vi "UHR-Fleezers Control (host) - 10.7.vi"() -> ()   [LabVIEW 2010] (continued)
        n1245 = event-data() -> ("CtlRef"=w4736:refnum<vi>)  [unwired: 6 out]
        n1246 = control-ref of="Trap Delta (MHz)"() -> (w4735:refnum<vi>)
        n1247 = Equal?(x=w4735, y=w4736) -> (x = y?=w4734:bool)
        n1248 = case shown="False" "Oscillate Set 2" {
          tunnel: w4739 -> [w4759 _]
          tunnel: [w4758 w4762] -> w4738
          tunnel: w4737 -> [w4757 w4762]
          tunnel: w4734 -> [w4742 _]
          frame False {
            n1249 = local read "BD 1 Frequency 2 (MHz)"() -> (w4746:dbl)
            n1250 = local read "BD 1 Frequency 1 (MHz)"() -> (w4744:dbl)
            n1251 = Subtract(x=w4746, y="Trap Delta (MHz)") -> (x-y=w4743:dbl)
            n1252 = Select(t=w4743, s=w4742, f=w4744) -> (s? t:f=w4741:dbl)
            n1253 = local read "Y RF Frequency Limits (MHz)"() -> (w4747:T16)
            n1254 = local read "X RF Frequency Limits (MHz)"() -> (w4748:T16)
            n1255 = local read "BD 1 Frequency 3 (MHz)"() -> (w4760:dbl)
            n1256 = local write "BD 1 Frequency 1 (MHz)"(w4741) -> ()
            n1257 = local read "BD 2 Frequency 1 (MHz)"() -> (w4751:dbl)
            n1258 = local read "BD 2 Frequency 2 (MHz)"() -> (w4750:dbl)
            n1259 = local read "BD 2 Frequency 3 (MHz)"() -> (w4761:dbl)
            n1260 = call "set RF board frequency - interlace.vi"("Board 2 Frequency Limits"=w4747, "Board 1 Frequency Limits"=w4748, "error in"=w4757, "FPGA VI Reference In"=w4759, "Board 2 Frequency 3 (MHz)"=w4761, "Board 1 Frequency 3 (MHz)"=w4760, "Board 2 Frequency 2 (MHz)"=w4750, "Board 2 Frequency 1 (MHz)"=w4751, "Board 1 Frequency 2 (MHz)"=w4746, "Board 1 Frequency 1  (MHz)"=w4741) -> ("error out"=w4758:errorcluster)  [unwired: 1 out]
            n1261 = Subtract(x=w4751, y=w4750) -> (x-y=w4755:dbl)
            n1262 = Subtract(x=w4741, y=w4746) -> (x-y=w4756:dbl)
            n1263 = Square(x=w4755) -> (x^2=w4753:dbl)
            n1264 = Square(x=w4756) -> (x^2=w4754:dbl)
            n1265 = Add(x=w4754, y=w4753) -> (x+y=w4752:dbl)
            n1266 = Square Root(x=w4752) -> (sqrt(x)=w4749:dbl)
            n1267 = local write "Trap Delta (MHz)"(w4749) -> ()
            n1268 = property on="Initial delta (MHz)" class="DigNum (strict)"("Val(Sgnl)"=w4749) -> ()  [unwired: 2 in, 2 out]
          }
          frame True {
          }
        }
      }
      event "Round T1 X": Value Change {
        n1269 = event-data() -> ()  [unwired: 7 out]
        n1270 = local read "BD 1 Frequency 1 (MHz)"() -> (w4765:dbl)
        n1271 = Round To Nearest(number=w4765) -> (nearest integer value=w4764:dbl)
        n1272 = property on="BD 1 Frequency 1 (MHz)" class="DigNum (strict)"("Val(Sgnl)"=w4764) -> ()  [unwired: 2 in, 2 out]
      }
      event "Restart RF": Value Change {
        n1273 = event-data() -> ()  [unwired: 7 out]
        n1274 = xnode "Read/Write Control"("FPGA VI Reference In"=w4803, "error in"=w4798, "FPGA Controls  RF Box"=FALSE) -> ("FPGA VI Reference Out"=w4802:T19, "error out"=w4797:errorcluster)
        n1275 = local read "Y RF Amplitude Limits (%)"() -> (w4778:T16)
        n1276 = local read "X RF Amplitude Limits (%)"() -> (w4779:T16)
        n1277 = local read "X RF Frequency Limits (MHz)"() -> (w4781:T16)
        n1278 = local read "Y RF Frequency Limits (MHz)"() -> (w4780:T16)
        n1279 = xnode "Read/Write Control"("FPGA VI Reference In"=w4802, "error in"=w4797, "Direct RF Box  Communication"=TRUE) -> ("FPGA VI Reference Out"=w4801:T19, "error out"=w4796:errorcluster)
        n1280 = local read "BD 2 Frequency 3 (MHz)"() -> (w4788:dbl)
        n1281 = local read "BD 2 Frequency 2 (MHz)"() -> (w4789:dbl)
        n1282 = local read "BD 1 Frequency 3 (MHz)"() -> (w4792:dbl)
        n1283 = local read "BD 1 Frequency 1 (MHz)"() -> (w4793:dbl)
        n1284 = local read "BD 2 Frequency 1 (MHz)"() -> (w4790:dbl)
        n1285 = local read "BD 1 Frequency 2 (MHz)"() -> (w4791:dbl)
        n1286 = call "Initialize RF boards - interlace 3.vi"("error in"=w4796, "FPGA VI Reference In"=w4801) -> ("error out"=w4795:errorcluster, "FPGA VI Reference Out"=w4800:T19)
        n1287 = local read "BD 2 Amplitude 2 (%)"() -> (w4783:dbl)
        n1288 = local read "BD 2 Amplitude 1 (%)"() -> (w4784:dbl)
        n1289 = local read "BD 2 Amplitude 3 (%)"() -> (w4782:dbl)
        n1290 = local read "BD 1 Amplitude 3 (%)"() -> (w4787:dbl)
        n1291 = local read "BD 1 Amplitude 1 (%)"() -> (w4786:dbl)
        n1292 = local read "BD 1 Amplitude 2 (%)"() -> (w4785:dbl)
        n1293 = call "set RF board frequency - interlace.vi"("Board 2 Frequency Limits"=w4780, "Board 1 Frequency Limits"=w4781, "error in"=w4795, "FPGA VI Reference In"=w4800, "Board 2 Frequency 3 (MHz)"=w4788, "Board 1 Frequency 3 (MHz)"=w4792, "Board 2 Frequency 2 (MHz)"=w4789, "Board 2 Frequency 1 (MHz)"=w4790, "Board 1 Frequency 2 (MHz)"=w4791, "Board 1 Frequency 1  (MHz)"=w4793) -> ("error out"=w4794:errorcluster, "FPGA VI Reference Out"=w4799:T19)
        n1294 = call "set RF board amplitude - interlace.vi"("Board 2 Amplitude Limits"=w4778, "Board 1 Amplitude Limits"=w4779, "error in"=w4794, "FPGA VI Reference In"=w4799, "Board 2 Amplitude 3 (%)"=w4782, "Board 1 Amplitude 3 (%)"=w4787, "Board 2 Amplitude 2 (%)"=w4783, "Board 2 Amplitude 1 (%)"=w4784, "Board 1 Amplitude 2 (%)"=w4785, "Board 1 Amplitude 1 (%)"=w4786) -> ("error out"=w4771:errorcluster, "FPGA VI Reference Out"=w4775:T19)
        n1295 = xnode "Read/Write Control"("FPGA VI Reference In"=w4775, "error in"=w4771, "Direct RF Box  Communication"=FALSE) -> ("FPGA VI Reference Out"=w4774:T19, "error out"=w4773:errorcluster)
        n1296 = flat-sequence {
          tunnel: w4773 -> [w4804]
          tunnel: [w4804] -> w4772
          frame #0 {
            n1297 = Wait (ms)(milliseconds to wait=u32 50) -> ()  [unwired: 1 out]
          }
        }
        n1298 = xnode "Read/Write Control"("FPGA VI Reference In"=w4774, "error in"=w4772, "FPGA Controls  RF Box"=TRUE) -> ("error out"=w4767:errorcluster)  [unwired: 1 out]
        n1299 = property on="Restart RF" class="Bool (strict)"(error in=w4767, "Value"=FALSE ("Restart RF")) -> (error out=w4766:errorcluster)  [unwired: 1 in, 1 out]
      }
      event "Round T2 X": Value Change {
        n1300 = event-data() -> ()  [unwired: 7 out]
        n1301 = local read "BD 1 Frequency 2 (MHz)"() -> (w4959:dbl)
        n1302 = Round To Nearest(number=w4959) -> (nearest integer value=w4958:dbl)
        n1303 = property on="BD 1 Frequency 2 (MHz)" class="DigNum (strict)"("Val(Sgnl)"=w4958) -> ()  [unwired: 2 in, 2 out]
      }
      event "Stop All": Value Change {
        n1304 = event-data() -> ()  [unwired: 7 out]
        n1305 = call "hamilton_controller.vi"("action"=T23."DISCONNECT") -> ()  [unwired: 10 in, 1 out]
        n1306 = local read "Stop All"() -> (w4962:bool)
      }
      event "Delayed Interlace Start": Value Change {
        n1307 = event-data() -> ()  [unwired: 7 out]
        n1308 = flat-sequence {
          frame #0 {
            n1309 = Multiply(x="Delay to Interlace (s)", y=1000.0) -> (x*y=w4965:dbl)
            n1310 = Wait (ms)(milliseconds to wait=w4965) -> ()  [unwired: 1 out]
          }
          frame #1 {
            n1311 = property on="Green laser mode" class="RadioBtnsControl (strict)"("Val(Sgnl)"=enum32{"Laser ON", "Laser OFF", "Interlace"}."Interlace" ("Value (Signaling)")) -> ()  [unwired: 2 in, 2 out]
          }
        }
      }
      event "BD 1 Amplitude 1 (%)", "BD 1 Amplitude 2 (%)", "BD 1 Amplitude 3 (%)", "BD 2 Amplitude 1 (%)", "BD 2 Amplitude 2 (%)", "BD 2 Amplitude 3 (%)", "Trap 1 ON", "Trap 2 ON", "Trap 3 ON", "Feedback On/Off", "All FB On/Off": Value Change {
        w4989 = i16 1 ("f")
        n1312 = event-data() -> ()  [unwired: 7 out]
        n1313 = local write "Trap 1 (ON/OFF)"("Trap 1 ON") -> ()
        n1314 = local write "Trap 2 (ON/OFF)"("Trap 2 ON") -> ()
        n1315 = Boolean To (0,1)(Boolean="Trap 3 ON") -> (0, 1=w4990:i16)
        n1316 = Boolean To (0,1)(Boolean="Trap 1 ON") -> (0, 1=w4991:i16)
        n1317 = Boolean To (0,1)(Boolean="Trap 2 ON") -> (0, 1=w4992:i16)
        n1318 = Select(t=w4992, s="Trap ON/OFF X or Y Amp?", f=w4989) -> (s? t:f=w4987:i16)
        n1319 = Select(t=w4991, s="Trap ON/OFF X or Y Amp?", f=w4989) -> (s? t:f=w4988:i16)
        n1320 = Select(t=w4990, s="Trap ON/OFF X or Y Amp?", f=w4989) -> (s? t:f=w4986:i16)
        n1321 = Select(t=w4989, s="Trap ON/OFF X or Y Amp?", f=w4992) -> (s? t:f=w4984:i16)
        n1322 = Select(t=w4989, s="Trap ON/OFF X or Y Amp?", f=w4991) -> (s? t:f=w4985:i16)
        n1323 = Select(t=w4989, s="Trap ON/OFF X or Y Amp?", f=w4990) -> (s? t:f=w4983:i16)
        n1324 = And(x="All FB On/Off", y="Feedback On/Off") -> (x .and. y?=w4981:cluster{"Set 1":bool, "Set 2":bool})
        n1325 = local read "BD 1 Amplitude 1 (%)"() -> (w5001:dbl)
        n1326 = local read "BD 1 Amplitude 2 (%)"() -> (w5000:dbl)
        n1327 = local read "BD 1 Amplitude 3 (%)"() -> (w4999:dbl)
        n1328 = Unbundle By Name(w4981) -> ("Set 1"=w4976:bool, "Set 2"=w4973:bool)
        n1329 = local read "Y RF Amplitude Limits (%)"() -> (w4969:T16)
        n1330 = local read "X RF Amplitude Limits (%)"() -> (w4970:T16)
        n1331 = local read "BD 2 Amplitude 1 (%)"() -> (w5002:dbl)
        n1332 = local read "BD 2 Amplitude 2 (%)"() -> (w5003:dbl)
        n1333 = local read "BD 2 Amplitude 3 (%)"() -> (w5004:dbl)
        n1334 = And(x="Trap 2 ON", y=w4973) -> (x .and. y?=w4971:bool)
        n1335 = And(x="Trap 1 ON", y=w4976) -> (x .and. y?=w4974:bool)
        n1336 = Multiply(x=w4988, y=w5001) -> (x*y=w4996:dbl)
        n1337 = Multiply(x=w5000, y=w4987) -> (x*y=w4994:dbl)
        n1338 = Multiply(x=w4999, y=w4986) -> (x*y=w4995:dbl)
        n1339 = Multiply(x=w5002, y=w4985) -> (x*y=w5005:dbl)
        n1340 = Multiply(x=w5003, y=w4984) -> (x*y=w5006:dbl)
        n1341 = Multiply(x=w5004, y=w4983) -> (x*y=w5007:dbl)
        n1342 = call "set RF board amplitude - interlace.vi"("Board 2 Amplitude Limits"=w4969, "Board 1 Amplitude Limits"=w4970, "error in"=w4997, "FPGA VI Reference In"=w4998, "Board 2 Amplitude 3 (%)"=w5007, "Board 1 Amplitude 3 (%)"=w4995, "Board 2 Amplitude 2 (%)"=w5006, "Board 2 Amplitude 1 (%)"=w5005, "Board 1 Amplitude 2 (%)"=w4994, "Board 1 Amplitude 1 (%)"=w4996) -> ("error out"=w4978:errorcluster, "FPGA VI Reference Out"=w4979:T19)
        n1343 = xnode "Read/Write Control"("FPGA VI Reference In"=w4979, "error in"=w4978, "FB On/Off Set 1"=w4974, "FB On/Off Set 2"=w4971) -> ("error out"=w4977:errorcluster)  [unwired: 1 out]
      }
      event "Load parameters": Value Change {
        n1344 = event-data() -> ()  [unwired: 7 out]
        n1345 = property on="Saved AOD Raster Scan Parameter Sets" class="Arr (strict)"() -> ("Index Values"=w5077:u32[])  [unwired: 2 in, 2 out]
        n1346 = Index Array(array=w5077, index=0) -> (element=w5074:u32)
        n1347 = local write "Load parameters"(FALSE ("Load parameters")) -> ()
        n1348 = Index Array(array="Saved AOD Raster Scan Parameter Sets", index=w5074) -> (element=w5073:T48)
        n1349 = Unbundle By Name(w5073) -> ("Scan Range AOD (nm) 2"=w5072:dbl, "Step Size AOD (nm) 2"=w5071:dbl, "Scan Speed AOD (nm/s) 2"=w5070:dbl, "Number of scans (AOD) 2"=w5069:u16)
        n1350 = flat-sequence {
          tunnel: w5072 -> [w5080]
          tunnel: w5071 -> [w5079]
          tunnel: w5070 -> [w5078]
          tunnel: w5069 -> [w5081]
          frame #0 {
            n1351 = local write "Scan Speed (nm/s)"(w5078) -> ()
            n1352 = local write "Scan Range (nm)"(w5080) -> ()
            n1353 = local write "Step Size (nm)"(w5079) -> ()
          }
          frame #1 {
            n1354 = property on="Number of F/B Scans (AOD)" class="DigNum (strict)"("Val(Sgnl)"=w5081) -> ()  [unwired: 2 in, 2 out]
          }
        }
      }
      event "Trap 1 (ON/OFF)", "Trap 2 (ON/OFF)": Value Change {
        n1355 = event-data() -> ()  [unwired: 7 out]
        n1356 = property on="Trap 2 ON" class="Bool (strict)"("Val(Sgnl)"="Trap 2 (ON/OFF)") -> ()  [unwired: 2 in, 2 out]
        n1357 = property on="Trap 1 ON" class="Bool (strict)"("Val(Sgnl)"="Trap 1 (ON/OFF)") -> ()  [unwired: 2 in, 2 out]
      }
      event "DIO count 1 (ticks)", "DIO count 2 (ticks)", "DIO count 3 (ticks)", "Interlace", "Number Interlace Sets", "Not-Interlacing Set": Value Change {
        n1358 = event-data() -> ()  [unwired: 7 out]
        n1359 = local read "DIO count 3 (ticks)"() -> (w5094:u32)
        n1360 = local read "DIO count 1 (ticks)"() -> (w5096:u32)
        n1361 = local read "DIO count 2 (ticks)"() -> (w5095:u32)
        n1362 = To Unsigned Byte Integer(number="Not-Interlacing Set") -> (unsigned 8bit integer=w5085:u8)
        n1363 = Add(x=w5085, y=u8 1) -> (x+y=w5089:u8)
        n1364 = xnode "Read/Write Control"("FPGA VI Reference In"=w5100, "error in"=w5098, "DIO count 1 (ticks)"=w5096, "DIO count 2 (ticks)"=w5095, "DIO count 3 (ticks)"=w5094, "Interlace ON/OFF"="Interlace", "Number Interlace Cycles"="Number Interlace Sets", "Interlace Off Parameters"=w5089) -> ("error out"=w5099:errorcluster)  [unwired: 1 out]
        n1365 = Build Array(w5096, w5095, w5094) -> (w5087:u32[])
        n1366 = Split 1D Array(array=w5087, index="Number Interlace Sets") -> (first subarray=w5097:u32[])  [unwired: 1 out]
        n1367 = Index Array(array=w5087, index=w5085) -> (element=w5086:u32)
        n1368 = Add Array Elements(numeric array=w5097) -> (sum=w5091:u32)
        n1369 = Select(t=w5091, s="Interlace", f=w5086) -> (s? t:f=→"Total Counts (ticks)":u32)
      }
      event "Reset Feedback": Value Change {
        n1370 = event-data() -> ()  [unwired: 7 out]
        n1371 = Unbundle By Name("Reset Feedback") -> ("Set 1"=w5242:bool, "Set 2"=w5241:bool)
        n1372 = xnode "Read/Write Control"("FPGA VI Reference In"=w5244, "error in"=w5239, "FB Reset Set 1"=w5242, "FB Reset Set 2"=w5241) -> ("error out"=w5240:errorcluster)  [unwired: 1 out]
      }
      event "PID Gains": Value Change {
        n1373 = event-data() -> ()  [unwired: 7 out]
        n1374 = Unbundle By Name("PID Gains") -> ("Set 1"=w5307:T14, "Set 2"=w5306:T14)
        n1375 = xnode "Read/Write Control"("FPGA VI Reference In"=w5308, "error in"=w5304, "FB Gains Set 1"=w5307, "FB Gains Set 2"=w5306) -> ("error out"=w5305:errorcluster)  [unwired: 1 out]
      }
      event "AI2 to Setpoint", "Trap Intensity\nSetpoints (V)": Value Change {
        n1376 = event-data() -> ()  [unwired: 7 out]
        n1377 = xnode "Read/Write Control"("FPGA VI Reference In"=w5383, "error in"=w5379) -> ("FPGA VI Reference Out"=w5382:T19, "error out"=w5381:errorcluster, "AI2 Y Sum Set 1"=w5390:i16, "AI2 Y Sum Set 2"=w5389:i16)
        n1378 = Cluster To Array(cluster="AI2 to Setpoint") -> (array=w5393:bool[])
        n1379 = local read "AI2 (V)"() -> (w5391:cluster{"Set 1":dbl, "Set 2":dbl})
        n1380 = Or Array Elements(Boolean array=w5393) -> (logical OR=w5394:bool)
        n1381 = Bundle By Name(cluster=w5391, "Set 1"=w5390, "Set 2"=w5389) -> (w5388:cluster{"Set 1":dbl, "Set 2":dbl})
        n1382 = Divide(x=w5388, y=3276.7) -> (x/y=w5387:cluster{"Set 1":dbl, "Set 2":dbl})
        "AI2 (V)" <- w5387
        n1383 = case shown="True" w5394 {
          tunnel: [w5458 w5475] -> w5386
          tunnel: "AI2 to Setpoint" -> [_ w5471]
          tunnel: "Trap Intensity\nSetpoints (V)" -> [w5459 w5474]
          tunnel: w5387 -> [_ w5468]
          frame False {
            n1384 = Multiply(x=3276.7, y=w5459) -> (x*y=w5460:cluster{"Set 1":dbl, "Set 2":dbl})
            n1385 = To Word Integer(number=w5460) -> (16bit integer=w5458:cluster{"Set 1":i16, "Set 2":i16})
          }
          frame True {
            n1386 = Unbundle By Name(w5468) -> ("Set 1"=w5467:dbl, "Set 2"=w5466:dbl)
            n1387 = Unbundle By Name(w5474) -> ("Set 1"=w5473:dbl, "Set 2"=w5472:dbl)
            n1388 = Unbundle By Name(w5471) -> ("Set 1"=w5470:bool, "Set 2"=w5469:bool)
            n1389 = Select(t=w5467, s=w5470, f=w5473) -> (s? t:f=w5465:dbl)
            n1390 = Select(t=w5466, s=w5469, f=w5472) -> (s? t:f=w5464:dbl)
            n1391 = Bundle By Name(cluster=w5474, "Set 1"=w5465, "Set 2"=w5464) -> (w5462:cluster{"Set 1":dbl, "Set 2":dbl})
            n1392 = local write "Trap Intensity\nSetpoints (V)"(w5462) -> ()
            n1393 = Multiply(x=3276.7, y=w5462) -> (x*y=w5463:cluster{"Set 1":dbl, "Set 2":dbl})
            n1394 = To Word Integer(number=w5463) -> (16bit integer=w5475:cluster{"Set 1":i16, "Set 2":i16})
          }
        }
        n1395 = Unbundle By Name(w5386) -> ("Set 1"=w5385:i16, "Set 2"=w5384:i16)
        n1396 = xnode "Read/Write Control"("FPGA VI Reference In"=w5382, "error in"=w5381, "FB Setpoint Set 1"=w5385, "FB Setpoint Set 2"=w5384) -> ("error out"=w5380:errorcluster)  [unwired: 1 out]
      }
      event "Invert GI": Value Change {
        n1397 = event-data() -> ()  [unwired: 7 out]
        n1398 = xnode "Read/Write Control"("FPGA VI Reference In"=w5537, "error in"=w5535, "Invert GI"="Invert GI", "Invert GI 2"="Invert GI") -> ("error out"=w5536:errorcluster)  [unwired: 1 out]
      }
      event "Green FB Setpoint (mV)", "Green FB Gains", "Green FB On/Off", "Current When FB OFF (%)", "Green int current ON count adj": Value Change {
        n1399 = event-data() -> ()  [unwired: 7 out]
        n1400 = local read "Green FB Setpoint (mV)"() -> (w5603:dbl)
        n1401 = local read "Current When FB OFF (%)"() -> (w5606:dbl)
        n1402 = Multiply(x=w5603, y=3.2767) -> (x*y=w5602:dbl)
        n1403 = Multiply(x=w5606, y=655.35) -> (x*y=w5607:dbl)
        n1404 = To Unsigned Word Integer(number=w5607) -> (unsigned 16bit integer=w5605:u16)
        n1405 = local read "Green int current ON count adj"() -> (w5610:u32)
        n1406 = local read "Green FB Gains"() -> (w5609:T14)
        n1407 = local read "Green Laser ON/Interlacing"() -> (w5600:bool)
        n1408 = local read "Green laser mode"() -> (w5599:enum32{"Laser ON", "Laser OFF", "Interlace"})
        n1409 = local read "Green FB On/Off"() -> (w5611:bool)
        n1410 = Equal?(x=w5599, y=enum32{"Laser ON", "Laser OFF", "Interlace"}."Interlace") -> (x = y?=w5597:bool)
        n1411 = Compound Arithmetic op=AND(w5597, w5611, w5600) -> (w5601:bool)
        n1412 = xnode "Read/Write Control"("FPGA VI Reference In"=w5614, "error in"=w5613, "Green FB Setpoint"=w5602, "Green FB On/Off"=w5601, "Current Out"=w5605, "Green int current ON count adj"=w5610, "Green FB Gains"=w5609) -> ("error out"=w5612:errorcluster)  [unwired: 1 out]
      }
      event "Green laser mode", "Green Laser ON/Interlacing": Value Change {
        n1413 = event-data() -> ()  [unwired: 7 out]
        n1414 = case shown="True" "Green Laser ON/Interlacing" {
          tunnel: "Green laser mode" -> [_ w5752]
          tunnel: [enum32{"Laser ON", "Laser OFF", "Interlace"}."Laser OFF" ("Green laser mode") w5752] -> w5740
          tunnel: [FALSE w5748] -> w5739
          frame False {
          }
          frame True {
            n1415 = local read "Green FB On/Off"() -> (w5749:bool)
            n1416 = Equal?(x=w5752, y=enum32{"Laser ON", "Laser OFF", "Interlace"}."Interlace") -> (x = y?=w5750:bool)
            n1417 = And(x=w5750, y=w5749) -> (x .and. y?=w5748:bool)
          }
        }
        n1418 = xnode "Read/Write Control"("FPGA VI Reference In"=w5745, "error in"=w5743, "Operating Mode"=w5740, "Operating Mode 2"=w5740, "Green FB On/Off"=w5739) -> ("error out"=w5744:errorcluster)  [unwired: 1 out]
      }
      event "Use mouse to move stage\n(press mouse wheel to quit)": Value Change {
        n1419 = event-data() -> ()  [unwired: 7 out]
      }
      event "- phase (APD 1 Gate)", "+ phase (APD 1 Gate)": Value Change {
        n1420 = event-data() -> ()  [unwired: 7 out]
        n1421 = local read "Phase Adj. (APD 1 Gate)"() -> (w5831:i16)
        n1422 = Negate(x=w5831) -> (-x=w5839:i16)
        n1423 = Select(t=w5839, s="- phase (APD 1 Gate)", f=w5831) -> (s? t:f=w5838:i16)
        n1424 = Or(x="- phase (APD 1 Gate)", y="+ phase (APD 1 Gate)") -> (x .or. y?=w5834:bool)
        n1425 = xnode "Read/Write Control"("FPGA VI Reference In"=w5841, "error in"=w5840, "Phase count adjustment (APD 1 Gate)"=w5838) -> ("FPGA VI Reference Out"=w5836:T19, "error out"=w5837:errorcluster)
        n1426 = xnode "Read/Write Control"("FPGA VI Reference In"=w5836, "error in"=w5837, "+ phase (APD 1 Gate)"=w5834) -> ("error out"=w5835:errorcluster)  [unwired: 1 out]
      }
      event "+ phase (APD 2 Gate)", "- phase (APD 2 Gate)": Value Change {
        n1427 = event-data() -> ()  [unwired: 7 out]
        n1428 = local read "Phase Adj. (APD 2 Gate)"() -> (w5917:i16)
        n1429 = Negate(x=w5917) -> (-x=w5925:i16)
        n1430 = Select(t=w5925, s="- phase (APD 2 Gate)", f=w5917) -> (s? t:f=w5924:i16)
        n1431 = Or(x="- phase (APD 2 Gate)", y="+ phase (APD 2 Gate)") -> (x .or. y?=w5920:bool)
        n1432 = xnode "Read/Write Control"("FPGA VI Reference In"=w5927, "error in"=w5926, "Phase count adjustment (APD 2 Gate)"=w5924) -> ("FPGA VI Reference Out"=w5922:T19, "error out"=w5923:errorcluster)
        n1433 = xnode "Read/Write Control"("FPGA VI Reference In"=w5922, "error in"=w5923, "+ phase (APD 2 Gate)"=w5920) -> ("error out"=w5921:errorcluster)  [unwired: 1 out]
      }
      event "Phase Adj. (APD Acq)", "+ phase (APD Acq)", "- phase (APD Acq)": Value Change {
        n1434 = event-data() -> ()  [unwired: 7 out]
        n1435 = local read "Phase Adj. (APD Acq)"() -> (w6005:i16)
        n1436 = Negate(x=w6005) -> (-x=w6011:i16)
        n1437 = Select(t=w6011, s="+ phase (APD Acq)", f=w6005) -> (s? t:f=w6010:i16)
        n1438 = Or(x="+ phase (APD Acq)", y="- phase (APD Acq)") -> (x .or. y?=w6006:bool)
        n1439 = xnode "Read/Write Control"("FPGA VI Reference In"=w6013, "error in"=w6012, "Phase Count Adjustment (APD Acq)"=w6010) -> ("FPGA VI Reference Out"=w6008:T19, "error out"=w6009:errorcluster)
        n1440 = xnode "Read/Write Control"("FPGA VI Reference In"=w6008, "error in"=w6009, "+ phase (APD Acq)"=w6006) -> ("error out"=w6007:errorcluster)  [unwired: 1 out]
      }
      event "Phase adj. (GI)", "+ phase (GI)", "- phase (GI)": Value Change {
        n1441 = event-data() -> ()  [unwired: 7 out]
        n1442 = Negate(x="Phase adj. (GI)") -> (-x=w6097:i16)
        n1443 = Select(t=w6097, s="+ phase (GI)", f="Phase adj. (GI)") -> (s? t:f=w6096:i16)
        n1444 = Or(x="+ phase (GI)", y="- phase (GI)") -> (x .or. y?=w6092:bool)
        n1445 = xnode "Read/Write Control"("FPGA VI Reference In"=w6099, "error in"=w6098, "Phase count adjustment (GI)"=w6096) -> ("FPGA VI Reference Out"=w6094:T19, "error out"=w6095:errorcluster)
        n1446 = xnode "Read/Write Control"("FPGA VI Reference In"=w6094, "error in"=w6095, "+ phase (GI)"=w6092) -> ("error out"=w6093:errorcluster)  [unwired: 1 out]
      }
      event "Phase adj. (GI) 2", "+ phase (GI) 2", "- phase (GI) 2": Value Change {
        n1447 = event-data() -> ()  [unwired: 7 out]
        n1448 = Negate(x="Phase adj. (GI) 2") -> (-x=w6183:i16)
        n1449 = Select(t=w6183, s="+ phase (GI) 2", f="Phase adj. (GI) 2") -> (s? t:f=w6182:i16)
        n1450 = Or(x="+ phase (GI) 2", y="- phase (GI) 2") -> (x .or. y?=w6178:bool)
        n1451 = xnode "Read/Write Control"("FPGA VI Reference In"=w6185, "error in"=w6184, "Phase count adjustment (GI) 2"=w6182) -> ("FPGA VI Reference Out"=w6180:T19, "error out"=w6181:errorcluster)
        n1452 = xnode "Read/Write Control"("FPGA VI Reference In"=w6180, "error in"=w6181, "+ phase (GI) 2"=w6178) -> ("error out"=w6179:errorcluster)  [unwired: 1 out]
      }
      event "Phase adj. (Green FB)", "- phase (Green FB)", "+ phase (Green FB)": Value Change {
        n1453 = event-data() -> ()  [unwired: 7 out]
        n1454 = Negate(x="Phase adj. (Green FB)") -> (-x=w6269:i16)
        n1455 = Select(t=w6269, s="+ phase (Green FB)", f="Phase adj. (Green FB)") -> (s? t:f=w6268:i16)
        n1456 = Or(x="+ phase (Green FB)", y="- phase (Green FB)") -> (x .or. y?=w6264:bool)
        n1457 = xnode "Read/Write Control"("FPGA VI Reference In"=w6271, "error in"=w6270, "Phase count adjustment (Green FB)"=w6268) -> ("FPGA VI Reference Out"=w6266:T19, "error out"=w6267:errorcluster)
        n1458 = xnode "Read/Write Control"("FPGA VI Reference In"=w6266, "error in"=w6267, "+ phase (Green FB)"=w6264) -> ("error out"=w6265:errorcluster)  [unwired: 1 out]
      }
      event "Invert APD Gate", "APD Gate ON Count", "APD Gate OFF Count", "APD Gate", "APD Integration Time (s)", "APD 1 AO Mult.", "APD 2 AO Mult.": Value Change {
        n1459 = event-data() -> ()  [unwired: 7 out]
        n1460 = local read "APD Integration Time (s)"() -> (w6347:dbl)
        n1461 = local read "APD Gate ON Count"() -> (w6360:u32)
        n1462 = local read "APD Gate OFF Count"() -> (w6359:u32)
        n1463 = local read "Invert APD Gate"() -> (w6361:bool)
        n1464 = local read "APD Gate"() -> (w6358:enum32{"ON", "OFF", "Interlace"})
        n1465 = Multiply(x=w6347, y=40000000.0) -> (x*y=w6356:dbl)
        n1466 = Reciprocal(x=w6347) -> (1/x=→"APD Acq Rate (Hz)":dbl)
        n1467 = To Unsigned Long Integer(number=w6356) -> (unsigned 32bit integer=w6355:u32)
        n1468 = local read "DMA Update Period (s)"() -> (w6348:dbl)
        n1469 = Divide(x=w6348, y=w6347) -> (x/y=w6351:dbl)
        n1470 = local read "APD 1 AO Mult."() -> (w6353:i16)
        n1471 = local read "APD 2 AO Mult."() -> (w6352:i16)
        n1472 = Multiply(x=2.0, y=w6351) -> (x*y=w6350:dbl)
        n1473 = local write "APD Samples/FIFO Acq."(w6351) -> ()
        n1474 = local write "APD Elements/DMA read"(w6350) -> ()
        n1475 = xnode "Read/Write Control"("FPGA VI Reference In"=w6364, "error in"=w6363, "Invert APD Gate"=w6361, "APD Gate ON Count"=w6360, "APD Gate OFF Count"=w6359, "APD Acq Rate Count"=w6355, "APD Gate Operating Mode"=w6358, "APD 1 AO scale factor"=w6353, "APD 2 AO scale factor"=w6352) -> ("error out"=w6362:errorcluster)  [unwired: 1 out]
      }
      event "GI Frequency, ON count", "Green FB Count", "GI Frequency, OFF count": Value Change {
        n1476 = event-data() -> ()  [unwired: 7 out]
        n1477 = xnode "Read/Write Control"("FPGA VI Reference In"=w6528, "error in"=w6526, "Green interlace ON count"="GI Frequency, ON count", "Green interlace OFF count"="GI Frequency, OFF count", "Green interlace ON count 2"="GI Frequency, ON count", "Green interlace OFF count 2"="GI Frequency, OFF count", "Green FB Count"="Green FB Count") -> ("error out"=w6527:errorcluster)  [unwired: 1 out]
      }
      event "Number of F/B Scans (AOD)", "Scan Speed (nm/s)", "Scan BD", "Initial delta (MHz)", "Step Size (nm)", "Scan Range (nm)": Value Change {
        w6707 = 123.0  # AOM cal (nm/MHz)
        n1478 = event-data() -> ()  [unwired: 7 out]
        n1479 = local read "BD 1 Frequency 1 (MHz)"() -> (w6690:dbl)
        n1480 = local read "AOM X Cal (nm/MHz)"() -> (w6682:dbl)
        n1481 = local read "X RF Frequency Limits (MHz)"() -> (w6694:T16)
        n1482 = local read "Y RF Frequency Limits (MHz)"() -> (w6691:T16)
        n1483 = local read "BD 2 Frequency 1 (MHz)"() -> (w6696:dbl)
        n1484 = Negate(x="Scan Range (nm)") -> (-x=w6660:dbl)
        n1485 = Divide(x=w6660, y=w6682) -> (x/y=w6664:dbl)
        n1486 = Select(t=w6694, s="Scan BD", f=w6691) -> (s? t:f=w6693:T16)
        n1487 = Select(t=w6690, s="Scan BD", f=w6696) -> (s? t:f=w6695:dbl)
        n1488 = Unbundle By Name(w6693) -> ("Maximum"=w6702:dbl, "Minimum"=w6701:dbl)
        n1489 = Add(x=w6664, y=w6695) -> (x+y=w6699:dbl)
        n1490 = Divide(x=w6660, y="Step Size (nm)") -> (x/y=w6679:dbl)
        n1491 = Divide(x="Step Size (nm)", y=w6682) -> (x/y=w6688:dbl)
        n1492 = Absolute Value(x=w6679) -> (abs(x)=w6663:dbl)
        n1493 = Sign(1:w6660) -> (0:w6661:dbl)
        n1494 = In Range and Coerce(upper limit=w6702, x=w6699, lower limit=w6701) -> (coerced(x)=w6698:dbl, In Range?=w6700:bool)
        n1495 = To Unsigned Quad Integer(1:w6663) -> (0:w6678:u64)
        "Scan steps (AOD)" <- w6678
        n1496 = call "IR AOM freq to word.vi"("Frequency In (MHz)"=w6688) -> ("Frequency Word Out (double)"=w6685:dbl)
        n1497 = Multiply(x=w6661, y=w6685) -> (x*y=w6662:dbl)
        n1498 = Subtract(x=w6699, y=w6698) -> (x-y=w6697:dbl)
        n1499 = To Quad Integer(1:w6662) -> (0:w6684:i64)
        "Incr. int (AOD)" <- w6684
        n1500 = Subtract(x=w6664, y=w6697) -> (x-y=w6683:dbl)
        "Scan Range (MHz)" <- w6683
        n1501 = Select(t=w6664, s=w6700, f=w6683) -> (s? t:f=w6703:dbl)
        n1502 = Multiply(x=w6683, y=w6682) -> (x*y=w6681:dbl)
        n1503 = Decrement(x=w6678) -> (x-1=w6731:u64)
        n1504 = Negate(x=w6681) -> (-x=w6677:dbl)
        n1505 = local write "Scan Range (nm)"(w6677) -> ()
        n1506 = Divide(x=w6703, y=w6731) -> (x/y=w6687:dbl)
        "Scan Increment (MHz)" <- w6687
        n1507 = call "IR AOM freq to word.vi"("Frequency In (MHz)"=w6687) -> ("Frequency Word Out (double)"=w6686:dbl)
        n1508 = Divide(x="Step Size (nm)", y="Scan Speed (nm/s)") -> (x/y=w6674:dbl)
        n1509 = To Quad Integer(1:w6686) -> ()  [unwired: 1 out]
        n1510 = local read "Number Interlace Sets"() -> (w6658:u8)
        n1511 = local read "AI Count (ticks)"() -> (w6659:u32)
        n1512 = local read "Total Counts (ticks)"() -> (w6657:u32)
        n1513 = local read "# Samples/trap"() -> (w6689:u32)
        n1514 = Multiply(x=w6659, y=w6658) -> (x*y=w6656:u32)
        n1515 = Divide(x=w6657, y=w6656) -> (x/y=w6655:dbl)
        n1516 = Select(t=w6690, s="Scan BD", f=w6696) -> (s? t:f=w6728:dbl)
        "Initial freq. (MHz)" <- w6728
        n1517 = Add(x=w6703, y=w6728) -> (x+y=→"Final freq. (MHz)":dbl)
        n1518 = Divide(x=w6657, y=40000000.0) -> (x/y=w6673:dbl)
        n1519 = Divide(x=w6674, y=w6673) -> (x/y=w6672:dbl)
        n1520 = To Unsigned Quad Integer(1:w6672) -> (0:w6647:u64)
        n1521 = Quotient & Remainder(x=w6647, y=u64 2) -> (x-y*floor(x/y)=w6651:u64)  [unwired: 1 out]
        n1522 = Equal?(x=w6651, y=u64 0) -> (x = y?=w6649:bool)
        n1523 = Decrement(x=w6647) -> (x-1=w6648:u64)
        n1524 = Select(t=w6647, s=w6649, f=w6648) -> (s? t:f=w6646:u64)
        "Cycles/step (AOD)" <- w6646
        n1525 = xnode "Read/Write Control"("FPGA VI Reference In"=w6739, "error in"=w6738, "Scan steps"=w6678, "Number of scans"="Number of F/B Scans (AOD)", "Cycles per step"=w6646, "Scan freq.  increment"=w6684, "Scan BD"="Scan BD") -> ("error out"=w6737:errorcluster)  [unwired: 1 out]
        n1526 = Multiply(x=w6678, y=w6646) -> (x*y=w6732:u64)
        n1527 = Multiply(x=w6732, y=u64 2) -> (x*y=w6654:u64)
        n1528 = Multiply(x=w6655, y=w6654) -> (x*y=w6653:dbl)
        "Data points/scan (f/b)" <- w6653
        n1529 = Multiply(x=w6653, y="Number of F/B Scans (AOD)") -> (x*y=w6735:dbl)
        "Data points/scans" <- w6735
        n1530 = Divide(x=w6735, y=w6689) -> (x/y=→"N sets should be saved":dbl)
        n1531 = Multiply(x=w6732, y=w6673) -> (x*y=w6671:dbl)
        "Time/Scan (s) (AOD)" <- w6671
        n1532 = Select(t=w6703, s="Scan BD", f=0.0) -> (s? t:f=w6729:dbl)
        n1533 = Select(t=0.0, s="Scan BD", f=w6703) -> (s? t:f=w6725:dbl)
        n1534 = local read "BD 2 Frequency 2 (MHz)"() -> (w6721:dbl)
        n1535 = local read "BD 1 Frequency 2 (MHz)"() -> (w6724:dbl)
        n1536 = Add(x=w6725, y=w6696) -> (x+y=w6722:dbl)
        n1537 = Add(x=w6690, y=w6729) -> (x+y=w6723:dbl)
        n1538 = Multiply(x=w6671, y=2.0) -> (x*y=w6670:dbl)
        n1539 = Multiply(x=w6670, y="Number of F/B Scans (AOD)") -> (x*y=w6667:dbl)
        n1540 = Divide(x=w6667, y=60.0) -> (x/y=→"Time to Finish All (min)":dbl)
        n1541 = Add(x="Trap 2 Bead Size (nm)", y="Trap 1 Bead Size (nm)") -> (x+y=w6711:dbl)
        n1542 = Divide(x=w6711, y=2.0) -> (x/y=w6705:dbl)
        n1543 = local read "Initial delta (MHz)"() -> (w6708:dbl)
        n1544 = Subtract(x=w6722, y=w6721) -> (x-y=w6719:dbl)
        n1545 = Subtract(x=w6723, y=w6724) -> (x-y=w6720:dbl)
        n1546 = Square(x=w6719) -> (x^2=w6718:dbl)
        n1547 = Square(x=w6720) -> (x^2=w6717:dbl)
        n1548 = Add(x=w6717, y=w6718) -> (x+y=w6716:dbl)
        n1549 = Square Root(x=w6716) -> (sqrt(x)=w6715:dbl)
        "Final delta (MHz)" <- w6715
        n1550 = Multiply(x=w6707, y=w6715) -> (x*y=w6714:dbl)
        n1551 = Multiply(x=w6708, y=w6707) -> (x*y=w6706:dbl)
        n1552 = Subtract(x=w6706, y=w6705) -> (x-y=→"Initial sep (nm)":dbl)
        n1553 = Subtract(x=w6714, y=w6705) -> (x-y=→"Final sep (nm)":dbl)
      }
      event "Freq or Amp switch first", "Swap F1 and F2", "Freq switch delay", "Amp switch delay": Value Change {
        n1554 = event-data() -> ()  [unwired: 7 out]
        n1555 = local read "Freq or Amp switch first"() -> (w6876:bool)
        n1556 = local read "Amp switch delay"() -> (w6877:u16)
        n1557 = local read "Freq switch delay"() -> (w6879:u16)
        n1558 = local read "Swap F1 and F2"() -> (w6878:bool)
        n1559 = xnode "Read/Write Control"("FPGA VI Reference In"=w6882, "error in"=w6881, "Freq switch delay"=w6879, "Swap F1 and F2"=w6878, "Amp switch delay"=w6877, "Freq or Amp switch first"=w6876) -> ("error out"=w6880:errorcluster)  [unwired: 1 out]
      }
      event "Scan steps (MCL)", "Number of scans (MCL)", "Scan Range (V)\n(of steps)", "2D or 1D Scan", "N APD Samp/step", "Fast Scan Dir", "Continuous MCL Scanning", "Scan lines (y)": Value Change {
        w6983 = 32767.0 ("y")
        n1560 = event-data() -> ()  [unwired: 7 out]
        n1561 = Select(t="Scan lines (y)", s="2D or 1D Scan", f="Number of scans (MCL)") -> (s? t:f=w6988:u64)
        n1562 = Decrement(x="Scan steps (MCL)") -> (x-1=w7004:u64)
        n1563 = Divide(x="Scan Range (V)\n(of steps)", y=w7004) -> (x/y=w7003:dbl)
        "Desired Scan Incr (V)" <- w7003
        n1564 = local read "APD Integration Time (s)"() -> (w6996:dbl)
        n1565 = Multiply(x=w7003, y=w6983) -> (x*y=w7012:dbl)
        n1566 = Divide(x=w7012, y=10.0) -> (x/y=w7002:dbl)
        "Desired incr (int)" <- w7002
        n1567 = local read "Update Count (MCL)"() -> (w7008:u32)
        n1568 = Round Toward -Infinity(1:w7002) -> (0:w7011:dbl)
        n1569 = To Word Integer(number=w7011) -> (16bit integer=w6986:i16)
        "Actual Incr. int (MCL)" <- w6986
        n1570 = Multiply(x=w6996, y=40000000.0) -> (x*y=w7009:dbl)
        n1571 = Divide(x=w7009, y=w7008) -> (x/y=w7007:dbl)
        n1572 = Multiply(x=i16 10, y=w6986) -> (x*y=w6984:i16)
        n1573 = Multiply(x="N APD Samp/step", y=w7007) -> (x*y=w7006:dbl)
        "Cycles/step (MCL)" <- w7006
        n1574 = Divide(x=w6984, y=w6983) -> (x/y=→"Actual MCL Inc (V)":dbl)
        n1575 = Multiply(x="N APD Samp/step", y="Scan steps (MCL)") -> (x*y=w6998:dbl)
        n1576 = local read "APD Samples/FIFO Acq."() -> (w6995:dbl)
        n1577 = Multiply(x=w6998, y=u64 2) -> (x*y=w6997:dbl)
        "Data points/scan (f+b)" <- w6997
        n1578 = Multiply(x=w6997, y=w6988) -> (x*y=w7015:dbl)
        "Data points/scans (MCL)" <- w7015
        n1579 = Multiply(x=w6996, y=w6997) -> (x*y=w6989:dbl)
        "Time/f+b scan (s) (MCL)" <- w6989
        n1580 = Divide(x=w7015, y=w6995) -> (x/y=→"N sets should be saved (MCL)":dbl)
        n1581 = Multiply(x=w6989, y=w6988) -> (x*y=→"Total Time (s)":dbl)
        n1582 = Not(x="Fast Scan Dir") -> (.not. x?=w6993:bool)
        n1583 = xnode "Read/Write Control"("FPGA VI Reference In"=w7019, "error in"=w7018, "Scan steps (MCL)"="Scan steps (MCL)", "Number of scans (MCL)"=w6988, "Cycles per step (MCL)"=w7006, "Scan freq.  increment (MCL)"=w6986, "1D or 2D Scan?"="2D or 1D Scan", "MCL Scan Axis"=w6993, "Cont. Scan (MCL)"="Continuous MCL Scanning") -> ("error out"=w7017:errorcluster)  [unwired: 1 out]
      }
      event Key Down {
        n1584 = event-data() -> ("VKey"=w7193:T49)  [unwired: 10 out]
        n1585 = local read "z nudge increment (um)"() -> (w7192:dbl)
        n1586 = case shown="\"F4\"" w7193 {
          tunnel: "lateral step size (mm)" -> [w7196 w7201 w7206 w7214 _ _ _ _ _ _ _ _ _ _ _ _ _ _ _ _ _ _ _ _ _ _ _ _ _ _ _ _ _ _ _ _ _ _ _ _ _ _ _ _ _ _ _ _ _ _ _ _ _ _ _ _]
          tunnel: w7192 -> [_ _ _ _ w7217 w7224 _ _ _ _ _ _ _ _ _ _ _ _ _ _ _ _ _ _ _ _ _ _ _ _ _ _ _ _ _ _ _ _ _ _ _ _ _ _ _ _ _ _ _ _ _ _ _ _ _ _]
          frame "Up" {
            w7198 = 0.0 ("element")
            n1587 = Negate(x=w7196) -> (-x=w7195:dbl)
            n1588 = Build Array(w7198, w7195, w7198) -> (w7197:dbl[])
            n1589 = call "CONEX_FUNCTIONAL_GLOBAL.vi"("Axis"=enum16{"X", "Y", "Z", "XY", "XZ", "YZ", "XYZ"}."Y", "Position"=w7197, "Command"=T22."REL MOVE") -> ()  [unwired: 6 in, 3 out]
          }
          frame "Down" {
            w7203 = 0.0 ("element")
            n1590 = Build Array(w7203, w7201, w7203) -> (w7202:dbl[])
            n1591 = call "CONEX_FUNCTIONAL_GLOBAL.vi"("Axis"=enum16{"X", "Y", "Z", "XY", "XZ", "YZ", "XYZ"}."Y", "Position"=w7202, "Command"=T22."REL MOVE") -> ()  [unwired: 6 in, 3 out]
          }
          frame "Left" {
            w7207 = 0.0 ("element")
            n1592 = Build Array(w7206, w7207, w7207) -> (w7208:dbl[])
            n1593 = call "CONEX_FUNCTIONAL_GLOBAL.vi"("Axis"=enum16{"X", "Y", "Z", "XY", "XZ", "YZ", "XYZ"}."X", "Position"=w7208, "Command"=T22."REL MOVE") -> ()  [unwired: 6 in, 3 out]
          }
          frame "Right" {
            w7212 = 0.0 ("element")
            n1594 = Negate(x=w7214) -> (-x=w7213:dbl)
            n1595 = Build Array(w7213, w7212, w7212) -> (w7211:dbl[])
            n1596 = call "CONEX_FUNCTIONAL_GLOBAL.vi"("Axis"=enum16{"X", "Y", "Z", "XY", "XZ", "YZ", "XYZ"}."X", "Position"=w7211, "Command"=T22."REL MOVE") -> ()  [unwired: 6 in, 3 out]
          }
          frame "PageUp" {
            w7221 = 0.0 ("element")
            n1597 = Divide(x=w7217, y=1000.0) -> (x/y=w7219:dbl)
            n1598 = Build Array(w7221, w7221, w7219) -> (w7220:dbl[])
            n1599 = call "CONEX_FUNCTIONAL_GLOBAL.vi"("Axis"=enum16{"X", "Y", "Z", "XY", "XZ", "YZ", "XYZ"}."Z", "Position"=w7220, "Command"=T22."REL MOVE") -> ()  [unwired: 6 in, 3 out]
          }
          frame "PageDown" {
            w7228 = 0.0 ("element")
            n1600 = Divide(x=w7224, y=-1000.0) -> (x/y=w7226:dbl)
            n1601 = Build Array(w7228, w7228, w7226) -> (w7227:dbl[])
            n1602 = call "CONEX_FUNCTIONAL_GLOBAL.vi"("Axis"=enum16{"X", "Y", "Z", "XY", "XZ", "YZ", "XYZ"}."Z", "Position"=w7227, "Command"=T22."REL MOVE") -> ()  [unwired: 6 in, 3 out]
          }
          frame Default {
          }
          frame "Insert" {
          }
          frame "Delete" {
          }
          frame "Home" {
          }
          frame "End" {
          }
          frame "Escape" {
          }
          frame "Help" {
          }
          frame "Pause" {
          }
          frame "ScrollLock" {
          }
          frame "F1" {
          }
          frame "F2" {
          }
          frame "F3" {
          }
          frame "F4" {
          }
          frame "F5" {
          }
          frame "F6" {
          }
          frame "F7" {
          }
          frame "F8" {
          }
          frame "F9" {
            n1603 = local read "Trap 1 (ON/OFF)"() -> (w7232:bool)
            n1604 = Not(x=w7232) -> (.not. x?=w7231:bool)
            n1605 = property on="Trap 1 (ON/OFF)" class="Bool (strict)"("Val(Sgnl)"=w7231) -> ()  [unwired: 2 in, 2 out]
          }
          frame "F10" {
            n1606 = local read "Trap 2 (ON/OFF)"() -> (w7234:bool)
            n1607 = Not(x=w7234) -> (.not. x?=w7233:bool)
            n1608 = property on="Trap 2 (ON/OFF)" class="Bool (strict)"("Val(Sgnl)"=w7233) -> ()  [unwired: 2 in, 2 out]
          }
          frame "F11" {
          }
          frame "F12" {
            n1609 = local read "Use mouse to move stage\n(press mouse wheel to quit)"() -> (w7236:bool)
            n1610 = Not(x=w7236) -> (.not. x?=w7235:bool)
            n1611 = case shown="False" w7235 {
              frame False {
                n1612 = flat-sequence {
                  frame #0 {
                    n1613 = dll-call lib="user32.dll" fn="ShowCursor" label="Call Library Function"("Enable"=1) -> ()  [unwired: 3 in, 4 out]
                  }
                  frame #1 {
                    n1614 = Wait (ms)(milliseconds to wait=u32 1000) -> ()  [unwired: 1 out]
                  }
                }
                n1615 = property class="VI"() -> ("Panel"=w7238:refnum<vi>)  [unwired: 2 in, 2 out]
                n1616 = property class="Pnl"(reference=w7238) -> ("Panes[]"=w7239:refnum<vi>[])  [unwired: 1 in, 2 out]
                n1617 = for {
                  tunnel: w7239 -> [w7243] mode=indexing
                  tunnel: T47."Always On" ("Horizontal Scrollbar Visibility") -> [w7244]
                  n1618 = property class="Pane"(reference=w7243, "HorizScrollbarVisibility"=w7244) -> (reference out=w7242:refnum<vi>)  [unwired: 1 in, 1 out]
                  n1619 = property class="Pane"(reference=w7242, "VertScrollbarVisibility"=w7244) -> ()  [unwired: 1 in, 2 out]
                }
              }
              frame True {
                n1620 = property class="VI"() -> ("Panel"=w7246:refnum<vi>)  [unwired: 2 in, 2 out]
                n1621 = property class="Pnl"(reference=w7246) -> ("Panes[]"=w7247:refnum<vi>[])  [unwired: 1 in, 2 out]
                n1622 = flat-sequence {
                  frame #0 {
                    n1623 = dll-call lib="user32.dll" fn="ShowCursor" label="Call Library Function"("Enable"=0) -> ()  [unwired: 3 in, 4 out]
                  }
                  frame #1 {
                    n1624 = Wait (ms)(milliseconds to wait=u32 1000) -> ()  [unwired: 1 out]
                  }
                }
                n1625 = for {
                  tunnel: w7247 -> [w7252] mode=indexing
                  tunnel: T47."Always Off" ("Horizontal Scrollbar Visibility") -> [w7250]
                  n1626 = property class="Pane"(reference=w7252, "HorizScrollbarVisibility"=w7250) -> (reference out=w7251:refnum<vi>)  [unwired: 1 in, 1 out]
                  n1627 = property class="Pane"(reference=w7251, "VertScrollbarVisibility"=w7250) -> ()  [unwired: 1 in, 2 out]
                }
              }
            }
            n1628 = local write "Use mouse to move stage\n(press mouse wheel to quit)"(w7235) -> ()
          }
          frame "F13" {
          }
          frame "F14" {
          }
          frame "F15" {
          }
          frame "F16" {
          }
          frame "F17" {
          }
          frame "F18" {
          }
          frame "F19" {
          }
          frame "F20" {
          }
          frame "F21" {
          }
          frame "F22" {
          }
          frame "F23" {
          }
          frame "F24" {
          }
          frame "Play" {
          }
          frame "VolumeUp" {
          }
          frame "VolumeDown" {
          }
          frame "Mute" {
          }
          frame "Two Byte Char" {
          }
          frame "Break" {
          }
          frame "Clear" {
          }
          frame "NumLock" {
          }
          frame "Caps" {
          }
          frame "Opt" {
          }
          frame "Cmd" {
          }
          frame "Alt" {
          }
          frame "Ctrl" {
          }
          frame "Shift" {
          }
          frame "Return" {
          }
          frame "Enter" {
          }
          frame "ASCII" {
          }
        }
      }
      event "Read Cal": Value Change {
        w7254 = 1000.0 ("y")
        n1629 = event-data() -> ()  [unwired: 7 out]
        n1630 = local read "Save file name"() -> (w7279:path)
        n1631 = local write "Read Cal"(FALSE ("Read Cal")) -> ()
        n1632 = Strip Path(path=w7279) -> (stripped path=w7278:path)  [unwired: 1 out]
        n1633 = Path To String(path=w7278) -> (string=w7277:string)
        n1634 = Concatenate Strings(w7277, "\\current.cal" ("string")) -> (w7275:string)
        n1635 = String To Path(string=w7275) -> (path=w7274:path)
        n1636 = Open/Create/Replace File(file path (use dialog)=w7274, operation (0:open)=T25."open", access (0:read/write)=enum16{"read/write", "read-only", "write-only"}."read-only") -> (refnum out=w7282:refnum<file>, error out=w7268:errorcluster)  [unwired: 1 in, 3 out]
        n1637 = Deny Access(4:w7268, 7:w7282) -> (0:w7267:errorcluster, 3:w7273:refnum<file>)  [unwired: 1 out]
        n1638 = Read from Binary File(5:0.0, 8:w7267, 9:T39."big-endian, network order" ("byte order (0:big-endian, network order)"), 10:-1 ("count (1)"), 11:w7273) -> (0:w7266:errorcluster, 2:w7264:dbl[], 3:w7269:refnum<file>)  [unwired: 2 out]
        n1639 = Array To Cluster(array=w7264) -> (cluster=w7263:T50)
        n1640 = Unbundle(w7263) -> ("[0]"=w7262:dbl, "[1]"=w7261:dbl, "[2]"=w7260:dbl, "[3]"=w7259:dbl, "[4]"=w7258:dbl, "[5]"=w7257:dbl)
        n1641 = Close File(refnum=w7269, error in=w7266) -> (error out=→"Read cal error":errorcluster)  [unwired: 1 out]
        n1642 = Multiply(x=w7257, y=w7254) -> (x*y=w7255:dbl)
        n1643 = local write "T2 kappa_x (pN/nm)"(w7259) -> ()
        n1644 = local write "T1 kappa_x (pN/nm)"(w7260) -> ()
        n1645 = local write "T1 alpha_x (nm/V)"(w7262) -> ()
        n1646 = local write "T2 alpha_x (nm/V)"(w7261) -> ()
        n1647 = Multiply(x=w7258, y=w7254) -> (x*y=w7256:dbl)
        n1648 = local write "T1 offset_x (mV)"(w7256) -> ()
        n1649 = local write "T2 offset_x (mV)"(w7255) -> ()
      }
      event "Abort MCL Scan": Value Change {
        n1650 = event-data() -> ()  [unwired: 7 out]
        n1651 = local write "MCL Scanning"(FALSE ("MCL Scanning")) -> ()
        n1652 = xnode "Read/Write Control"("FPGA VI Reference In"=w7287, "error in"=w7286, "Abort scan (MCL)"="Abort MCL Scan") -> ("error out"=w7285:errorcluster)  [unwired: 1 out]
      }
      event "Update Count (MCL)": Value Change {
        n1653 = event-data() -> ()  [unwired: 7 out]
        n1654 = xnode "Read/Write Control"("FPGA VI Reference In"=w7329, "error in"=w7328, "MCL count"="Update Count (MCL)") -> ("error out"=w7327:errorcluster)  [unwired: 1 out]
      }
      event "Phase adjust (MCL)", "+ phase (MCL)", "- phase (MCL)": Value Change {
        n1655 = event-data() -> ()  [unwired: 7 out]
        n1656 = Negate(x="Phase adjust (MCL)") -> (-x=w7375:i16)
        n1657 = Select(t=w7375, s="- phase (MCL)", f="Phase adjust (MCL)") -> (s? t:f=w7373:i16)
        n1658 = Or(x="- phase (MCL)", y="+ phase (MCL)") -> (x .or. y?=w7368:bool)
        n1659 = xnode "Read/Write Control"("FPGA VI Reference In"=w7377, "error in"=w7376, "Phase count adjustment (MCL)"=w7373) -> ("FPGA VI Reference Out"=w7369:T19, "error out"=w7370:errorcluster)
        n1660 = xnode "Read/Write Control"("FPGA VI Reference In"=w7369, "error in"=w7370, "+ phase (MCL)"=w7368) -> ("error out"=w7367:errorcluster)  [unwired: 1 out]
      }
      event "Abort AOD Scan": Value Change {
        n1661 = event-data() -> ()  [unwired: 7 out]
        n1662 = xnode "Read/Write Control"("FPGA VI Reference In"=w7456, "error in"=w7455, "Abort scan"="Abort AOD Scan") -> ("error out"=w7454:errorcluster)  [unwired: 1 out]
      }
      event "Continuous AOD Scanning": Value Change {
        n1663 = event-data() -> ()  [unwired: 7 out]
        n1664 = xnode "Read/Write Control"("FPGA VI Reference In"=w7498, "error in"=w7497, "Cont. Scan"="Continuous AOD Scanning") -> ("error out"=w7496:errorcluster)  [unwired: 1 out]
      }
      event "Index": Value Change {
        n1665 = event-data() -> ()  [unwired: 7 out]
        n1666 = call "Create new save file.vi"("Insert"="", "Ext"=".dat" ("string"), "Index In"="Index") -> ("Path Out"=→"Save file name":path, "Index Out"=w7537:dbl)
        "Save index" <- w7537
        n1667 = local write "Index"(w7537) -> ()
      }
      event "AO1", "AO2": Value Change {
        w7552 = 10.0 ("y")
        w7551 = 32767.0 ("y")
        n1668 = event-data() -> ()  [unwired: 7 out]
        n1669 = local read "AO2"() -> (w7550:dbl)
        n1670 = local read "AO1"() -> (w7547:dbl)
        n1671 = Multiply(x=w7547, y=w7551) -> (x*y=w7546:dbl)
        n1672 = Multiply(x=w7550, y=w7551) -> (x*y=w7549:dbl)
        n1673 = Divide(x=w7546, y=w7552) -> (x/y=w7545:dbl)
        n1674 = Divide(x=w7549, y=w7552) -> (x/y=w7548:dbl)
        n1675 = To Word Integer(number=w7545) -> (16bit integer=w7553:i16)
        n1676 = To Word Integer(number=w7548) -> (16bit integer=w7554:i16)
        n1677 = xnode "Read/Write Control"("FPGA VI Reference In"=w7544, "error in"=w7543, "AO1"=w7553, "AO2"=w7554) -> ("error out"=w7542:errorcluster)  [unwired: 1 out]
      }
      event "Inject Bottom": Value Change {
        n1678 = event-data() -> ()  [unwired: 7 out]
        n1679 = disable-structure shown="Enabled" {
          disable-tunnel: "Inject Bottom" -> [w7613 w7653]
          frame Disabled {
            n1680 = local read "Chemyx Syringe Pump Serial Port"() -> (w7614:refnum<visa-resource-name>)
            n1681 = local read "Pump write delay (ms)"() -> (w7615:dbl)
            n1682 = case shown="True" w7613 {
              tunnel: w7615 -> [w7621 w7635]
              tunnel: w7614 -> [w7618 w7634]
              frame False {
                n1683 = flat-sequence {
                  tunnel: w7618 -> [w7622]
                  tunnel: [w7622] -> w7619
                  tunnel: w7621 -> [_]
                  tunnel: [w7625] -> w7620
                  tunnel: w7619 -> [w7625]
                  tunnel: w7620 -> [w7626]
                  tunnel: [w7626] -> w7616
                  tunnel: [w7628] -> w7617
                  tunnel: w7616 -> [w7628]
                  tunnel: w7617 -> [w7630]
                  frame #0 {
                    n1684 = call "Write to pump.vi"("string"="enter pump1", "VISA resource name"=w7622) -> ()  [unwired: 1 out]
                  }
                  frame #1 {
                    n1685 = Wait (ms)(milliseconds to wait="Pump pause delay (ms)") -> ()  [unwired: 1 out]
                  }
                  frame #2 {
                    n1686 = call "Write to pump.vi"("string"="stop", "VISA resource name"=w7626) -> ()  [unwired: 1 out]
                  }
                  frame #3 {
                    n1687 = Wait (ms)(milliseconds to wait=u32 500) -> ()  [unwired: 1 out]
                  }
                  frame #4 {
                    n1688 = call "Write to pump.vi"("string"="stop", "VISA resource name"=w7630) -> ()  [unwired: 1 out]
                  }
                }
              }
              frame True {
                n1689 = flat-sequence {
                  tunnel: w7634 -> [w7644]
                  tunnel: w7635 -> [w7639]
                  tunnel: w7635 -> [w7646]
                  tunnel: w7634 -> [w7647]
                  tunnel: [w7647] -> w7632
                  tunnel: [w7649] -> w7633
                  tunnel: w7632 -> [w7649]
                  tunnel: w7633 -> [w7651]
                  frame #0 {
                    n1690 = local read "All Pump Parameters"() -> (w7638:T5)
                    n1691 = Unbundle By Name(w7638) -> ("Pump 1"=w7645:T51)
                    n1692 = call "Set pump parameters.vi"("Pump write delay (ms)"=w7639, "Volume (uL)"="Ch 2 Inject Volume (uL)", "Rate (uL/h)"="Ch 1 Inject Rate (ul/h)", "Units"=4.0, "Pump #"=1.0, "Pump Parameters In"=w7645, "VISA resource name"=w7644) -> ("Pump Parameters Out"=w7637:T51)  [unwired: 3 in]
                    n1693 = Bundle By Name(cluster=w7638, "Pump 1"=w7637) -> (w7636:T5)
                    n1694 = local write "All Pump Parameters"(w7636) -> ()
                  }
                  frame #1 {
                    n1695 = Wait (ms)(milliseconds to wait=w7646) -> ()  [unwired: 1 out]
                  }
                  frame #2 {
                    n1696 = call "Write to pump.vi"("string"="start", "VISA resource name"=w7647) -> ()  [unwired: 1 out]
                  }
                  frame #3 {
                    n1697 = Wait (ms)(milliseconds to wait=u32 500) -> ()  [unwired: 1 out]
                  }
                  frame #4 {
                    n1698 = call "Write to pump.vi"("string"="start", "VISA resource name"=w7651) -> ()  [unwired: 1 out]
                  }
                }
              }
            }
          }
          frame Enabled {
            n1699 = call "hamilton_controller.vi"("Open?"=w7653, "valve"=enum16{"A", "B", "C", "D", "ALL"}."B", "action"=T23."MOVE VALVE") -> ()  [unwired: 8 in, 1 out]
          }
        }
      }
      event "Inject Top": Value Change {
        n1700 = event-data() -> ()  [unwired: 7 out]
        n1701 = disable-structure shown="Enabled" {
          disable-tunnel: "Inject Top" -> [_ w7697]
          frame Disabled {
            n1702 = local read "Pump write delay (ms)"() -> (w7658:dbl)